vi "3kButtonsSys36x36.vi"() -> ()   [LabVIEW 2011]
doc: "3000 buttons from haobo.li@pansino.com.cn\nhttp://www.linkedin.com/pub/haobo-li/17/8a/220\nthanks to\nhttp://www.fatcow.com/free-icons"
panel:
  in  "Pansino 2":bool
  in  "Pansino":bool
  in  "zootool":bool
  in  "zoom_selection":bool
  in  "zoom_refresh":bool
  in  "zoom_out":bool
  in  "zoom_layer":bool
  in  "zoom_last":bool
  in  "zoom_in":bool
  in  "zoom_fit":bool
  in  "zoom_extend":bool
  in  "zoom_actual_equal":bool
  in  "zoom_actual":bool
  in  "zoom":bool
  in  "youtube":bool
  in  "yelp":bool
  in  "yellow_submarine":bool
  in  "yahoo_messenger":bool
  in  "yacht":bool
  in  "xing":bool
  in  "xhtml_valid":bool
  in  "xhtml_go":bool
  in  "xhtml_delete":bool
  in  "xhtml_add":bool
  in  "xhtml":bool
  in  "x_ray":bool
  in  "www_page":bool
  in  "wrench_orange":bool
  in  "wrench":bool
  in  "wrapping_tight":bool
  in  "wrapping_square":bool
  in  "wrapping_magazine":bool
  in  "wrapping_inline":bool
  in  "wrapping_in_front":bool
  in  "wrapping_edit":bool
  in  "wrapping_between":bool
  in  "wrapping_behind":bool
  in  "world_link":bool
  in  "world_go":bool
  in  "world_edit":bool
  in  "world_delete":bool
  in  "world_add":bool
  in  "world":bool
  in  "workspace":bool
  in  "wordpress_blog":bool
  in  "wordpress":bool
  in  "wizard_women":bool
  in  "wizard":bool
  in  "wishlist_add":bool
  in  "winrar_view":bool
  in  "winrar_extract":bool
  in  "winrar_add":bool
  in  "wine_pairings":bool
  in  "windy":bool
  in  "widgets":bool
  in  "widescreen":bool
  in  "whistle":bool
  in  "weight":bool
  in  "weighing_mashine":bool
  in  "webcam_error":bool
  in  "webcam_delete":bool
  in  "webcam_add":bool
  in  "webcam":bool
  in  "web_concierge":bool
  in  "weather_sun":bool
  in  "weather_snow":bool
  in  "weather_rain":bool
  in  "weather_lightning":bool
  in  "weather_cloudy":bool
  in  "weather_clouds":bool
  in  "wand":bool
  in  "wallet":bool
  in  "walk":bool
  in  "vslider":bool
  in  "vrule":bool
  in  "vlc":bool
  in  "visa_electron":bool
  in  "visa_2":bool
  in  "visa":bool
  in  "virus_protection":bool
  in  "virb":bool
  in  "vimeo":bool
  in  "viewstack":bool
  in  "videodisplay":bool
  in  "video_mode":bool
  in  "video":bool
  in  "viddler":bool
  in  "vhs":bool
  in  "vector_delete":bool
  in  "vector_add":bool
  in  "vector":bool
  in  "vdividedbox":bool
  in  "vcard_edit":bool
  in  "vcard_delete":bool
  in  "vcard_add":bool
  in  "vcard":bool
  in  "vbox":bool
  in  "user_zorro":bool
  in  "user_yoda":bool
  in  "user_wicket":bool
  in  "user_waiter_female_black":bool
  in  "user_waiter_female":bool
  in  "user_waiter":bool
  in  "user_viking_female":bool
  in  "user_viking":bool
  in  "user_vietnamese_female":bool
  in  "user_vietnamese":bool
  in  "user_trooper_captain":bool
  in  "user_trooper":bool
  in  "user_swimmer_female":bool
  in  "user_swimmer_black":bool
  in  "user_swimmer":bool
  in  "user_superman":bool
  in  "user_suit":bool
  in  "user_student_female_black":bool
  in  "user_student_female":bool
  in  "user_student_black":bool
  in  "user_student":bool
  in  "user_striper_black":bool
  in  "user_striper":bool
  in  "user_stewardess_black":bool
  in  "user_stewardess":bool
  in  "user_squidward":bool
  in  "user_sponge_bob":bool
  in  "user_spiderman":bool
  in  "user_soldier":bool
  in  "user_silhouette":bool
  in  "user_scream":bool
  in  "user_samurai":bool
  in  "user_sailor_black":bool
  in  "user_sailor":bool
  in  "user_robocop":bool
  in  "user_redskin":bool
  in  "user_red":bool
  in  "user_rambo":bool
  in  "user_racer":bool
  in  "user_r2d2":bool
  in  "user_queen_black":bool
  in  "user_queen":bool
  in  "user_pumpkin":bool
  in  "user_priest_black":bool
  in  "user_priest":bool
  in  "user_policeman_black":bool
  in  "user_policeman":bool
  in  "user_police_female_black":bool
  in  "user_police_female":bool
  in  "user_police_england":bool
  in  "user_plankton":bool
  in  "user_pirate":bool
  in  "user_pilot_civil":bool
  in  "user_pilot":bool
  in  "user_patrick":bool
  in  "user_orange":bool
  in  "user_oldwoman_black":bool
  in  "user_oldwoman":bool
  in  "user_oldman_black":bool
  in  "user_oldman":bool
  in  "user_officer_black":bool
  in  "user_officer":bool
  in  "user_nun_black":bool
  in  "user_nun":bool
  in  "user_nude_female_black":bool
  in  "user_nude_female":bool
  in  "user_nude_black":bool
  in  "user_nude":bool
  in  "user_ninja":bool
  in  "user_muslim_female":bool
  in  "user_muslim":bool
  in  "user_mexican":bool
  in  "user_medical_female_black":bool
  in  "user_medical_female":bool
  in  "user_medical_black":bool
  in  "user_medical":bool
  in  "user_maid":bool
  in  "user_lisa":bool
  in  "user_leprechaun":bool
  in  "user_knight":bool
  in  "user_king_black":bool
  in  "user_king":bool
  in  "user_judge_black":bool
  in  "user_judge":bool
  in  "user_jew":bool
  in  "user_jester":bool
  in  "user_jawa":bool
  in  "user_jason":bool
  in  "user_ironman":bool
  in  "user_indian_female":bool
  in  "user_indian":bool
  in  "user_imprisoned_female_black":bool
  in  "user_imprisoned_female":bool
  in  "user_imprisoned_black":bool
  in  "user_imprisoned":bool
  in  "user_hendrix":bool
  in  "user_halk":bool
  in  "user_green":bool
  in  "user_gray":bool
  in  "user_goth":bool
  in  "user_gomer":bool
  in  "user_go":bool
  in  "user_gladiator":bool
  in  "user_geisha":bool
  in  "user_freddy":bool
  in  "user_firefighter_black":bool
  in  "user_firefighter":bool
  in  "user_female":bool
  in  "user_eskimo_female":bool
  in  "user_eskimo":bool
  in  "user_emo":bool
  in  "user_egyptian_female":bool
  in  "user_egyptian":bool
  in  "user_edit":bool
  in  "user_dracula":bool
  in  "user_diver":bool
  in  "user_devil":bool
  in  "user_detective_gray":bool
  in  "user_detective":bool
  in  "user_delete":bool
  in  "user_death":bool
  in  "user_darth_vader":bool
  in  "user_crabs":bool
  in  "user_cowboy_female":bool
  in  "user_cowboy":bool
  in  "user_cook_female_black":bool
  in  "user_cook_female":bool
  in  "user_cook_black":bool
  in  "user_cook":bool
  in  "user_comment":bool
  in  "user_clown":bool
  in  "user_chief_female_black":bool
  in  "user_chief_female":bool
  in  "user_chief_black":bool
  in  "user_chief":bool
  in  "user_catwomen":bool
  in  "user_c3po":bool
  in  "user_buddhist":bool
  in  "user_boxer_black":bool
  in  "user_boxer":bool
  in  "user_blondy":bool
  in  "user_bishop":bool
  in  "user_bender":bool
  in  "user_beach_lifeguard_female":bool
  in  "user_beach_lifeguard":bool
  in  "user_batman":bool
  in  "user_bart":bool
  in  "user_banker":bool
  in  "user_ballplayer_black":bool
  in  "user_ballplayer":bool
  in  "user_astronaut":bool
  in  "user_angel_female_black":bool
  in  "user_angel_female":bool
  in  "user_angel_black":bool
  in  "user_angel":bool
  in  "user_alien":bool
  in  "user_add":bool
  in  "user":bool
  in  "usb_3":bool
  in  "update":bool
  in  "universal_binary":bool
  in  "unicorn":bool
  in  "understanding":bool
  in  "underle_dictionary":bool
  in  "umbrella":bool
  in  "ufo":bool
  in  "ubuntu":bool
  in  "twitter_2":bool
  in  "twitter_1":bool
  in  "tux":bool
  in  "turntable":bool
  in  "tumblr":bool
  in  "tubes":bool
  in  "tub":bool
  in  "trolley":bool
  in  "trojan_horse":bool
  in  "tree":bool
  in  "travel":bool
  in  "transmit_go":bool
  in  "transmit_error":bool
  in  "transmit_edit":bool
  in  "transmit_delete":bool
  in  "transmit_blue":bool
  in  "transmit_add":bool
  in  "transmit":bool
  in  "transform_shear":bool
  in  "transform_selection":bool
  in  "transform_scale":bool
  in  "transform_rotate_270":bool
  in  "transform_rotate_180":bool
  in  "transform_rotate_90":bool
  in  "transform_rotate":bool
  in  "transform_perspective":bool
  in  "transform_path":bool
  in  "transform_move":bool
  in  "transform_layer":bool
  in  "transform_flip":bool
  in  "transform_crop_resize":bool
  in  "transform_crop":bool
  in  "traffic_usage":bool
  in  "traffic_lights_yellow":bool
  in  "traffic_lights_red":bool
  in  "traffic_lights_green":bool
  in  "traffic_lights":bool
  in  "trade":bool
  in  "tractor":bool
  in  "toxic":bool
  in  "tower":bool
  in  "toucan":bool
  in  "total_plan_cost":bool
  in  "toster":bool
  in  "tornado":bool
  in  "torchere":bool
  in  "tooth":bool
  in  "toolbox":bool
  in  "to_do_list_cheked_all":bool
  in  "to_do_list_cheked_1":bool
  in  "to_do_list":bool
  in  "title_window":bool
  in  "tire":bool
  in  "tipper":bool
  in  "timeline_marker":bool
  in  "timeline":bool
  in  "time_go":bool
  in  "time_delete":bool
  in  "time_add":bool
  in  "time":bool
  in  "tilelist":bool
  in  "tick":bool
  in  "thumb_up":bool
  in  "thumb_down":bool
  in  "three_tags":bool
  in  "things_digital":bool
  in  "things_beauty":bool
  in  "theater":bool
  in  "textfield_rename":bool
  in  "textfield_key":bool
  in  "textfield_delete":bool
  in  "textfield_add":bool
  in  "textfield":bool
  in  "text_width":bool
  in  "text_uppercase":bool
  in  "text_underline":bool
  in  "text_superscript":bool
  in  "text_subscript":bool
  in  "text_strikethroungh":bool
  in  "text_smallcaps":bool
  in  "text_signature":bool
  in  "text_resize":bool
  in  "text_replace":bool
  in  "text_prose":bool
  in  "text_pagination_100":bool
  in  "text_pagination":bool
  in  "text_padding_top":bool
  in  "text_padding_right":bool
  in  "text_padding_left":bool
  in  "text_padding_bottom":bool
  in  "text_lowercase":bool
  in  "text_list_numbers":bool
  in  "text_list_bullets":bool
  in  "text_linespacing":bool
  in  "text_letterspacing":bool
  in  "text_letter_omega":bool
  in  "text_large_cap":bool
  in  "text_language":bool
  in  "text_kerning":bool
  in  "text_italic":bool
  in  "text_indent_remove":bool
  in  "text_indent":bool
  in  "text_horizontalrule":bool
  in  "text_heading_6":bool
  in  "text_heading_5":bool
  in  "text_heading_4":bool
  in  "text_heading_3":bool
  in  "text_heading_2":bool
  in  "text_heading_1":bool
  in  "text_dropcaps":bool
  in  "text_drama":bool
  in  "text_document_wrap":bool
  in  "text_document":bool
  in  "text_columns":bool
  in  "text_bold":bool
  in  "text_area":bool
  in  "text_allcaps":bool
  in  "text_align_right":bool
  in  "text_align_left":bool
  in  "text_align_justity":bool
  in  "text_align_center":bool
  in  "text":bool
  in  "terminal_seats_red":bool
  in  "terminal_seats_blue":bool
  in  "terminal":bool
  in  "temperature_5":bool
  in  "temperature_4":bool
  in  "temperature_3":bool
  in  "temperature_2":bool
  in  "temperature_1":bool
  in  "television_delete":bool
  in  "television_add":bool
  in  "television":bool
  in  "telephone_link":bool
  in  "telephone_key":bool
  in  "telephone_go":bool
  in  "telephone_error":bool
  in  "telephone_edit":bool
  in  "telephone_delete":bool
  in  "telephone_add":bool
  in  "telephone":bool
  in  "teddy_bear":bool
  in  "technorati":bool
  in  "teapot":bool
  in  "tea_cup":bool
  in  "tags_cloud":bool
  in  "tag_yellow":bool
  in  "tag_red":bool
  in  "tag_purple":bool
  in  "tag_pink":bool
  in  "tag_orange":bool
  in  "tag_green":bool
  in  "tag_blue_edit":bool
  in  "tag_blue_delete":bool
  in  "tag_blue_add":bool
  in  "tag_blue":bool
  in  "tag":bool
  in  "tabnavigator":bool
  in  "tablets":bool
  in  "table_torn":bool
  in  "table_tab_search":bool
  in  "table_tab_resize":bool
  in  "table_tab":bool
  in  "table_sum":bool
  in  "table_split":bool
  in  "table_sort":bool
  in  "table_sheet":bool
  in  "table_select_row":bool
  in  "table_select_column":bool
  in  "table_select_big":bool
  in  "table_select_all":bool
  in  "table_select":bool
  in  "table_save":bool
  in  "table_row_insert":bool
  in  "table_row_delete":bool
  in  "table_replace":bool
  in  "table_relationship":bool
  in  "table_refresh":bool
  in  "table_paint_can":bool
  in  "table_multiple":bool
  in  "table_money":bool
  in  "table_link":bool
  in  "table_lightning":bool
  in  "table_key":bool
  in  "table_insert":bool
  in  "table_import":bool
  in  "table_heatmap":bool
  in  "table_go":bool
  in  "table_gear":bool
  in  "table_export":bool
  in  "table_excel":bool
  in  "table_error":bool
  in  "table_edit":bool
  in  "table_delete":bool
  in  "table_chart":bool
  in  "table_add":bool
  in  "table":bool
  in  "tabbar":bool
  in  "tab_go":bool
  in  "tab_edit":bool
  in  "tab_delete":bool
  in  "tab_add":bool
  in  "tab":bool
  in  "system_time":bool
  in  "system_monitor":bool
  in  "sword":bool
  in  "switch_220v":bool
  in  "switch_120v":bool
  in  "switch":bool
  in  "swf_loader":bool
  in  "support":bool
  in  "sun_rain":bool
  in  "sun_cloudy":bool
  in  "sum":bool
  in  "subwoofer":bool
  in  "style_go":bool
  in  "style_edit":bool
  in  "style_delete":bool
  in  "style_add":bool
  in  "style":bool
  in  "stumble_upon":bool
  in  "street_stall":bool
  in  "storage":bool
  in  "stopwatch_start":bool
  in  "stopwatch_pause":bool
  in  "stopwatch_finish":bool
  in  "stop":bool
  in  "stethoscope_vintage":bool
  in  "stethoscope":bool
  in  "steering_wheel_3":bool
  in  "steering_wheel_2":bool
  in  "steering_wheel":bool
  in  "steak_meat":bool
  in  "steak_fish":bool
  in  "status_online":bool
  in  "status_offline":bool
  in  "status_busy":bool
  in  "status_away":bool
  in  "statistics":bool
  in  "star":bool
  in  "stamp_pattern":bool
  in  "ssl_certificates":bool
  in  "sql_join_right_exclude":bool
  in  "sql_join_right":bool
  in  "sql_join_outer_exclude":bool
  in  "sql_join_outer":bool
  in  "sql_join_left_exclude":bool
  in  "sql_join_left":bool
  in  "sql_join_inner":bool
  in  "sql_join":bool
  in  "spring":bool
  in  "sport_tennis":bool
  in  "sport_soccer":bool
  in  "sport_shuttlecock":bool
  in  "sport_raquet":bool
  in  "sport_golf":bool
  in  "sport_football":bool
  in  "sport_basketball":bool
  in  "sport_8ball":bool
  in  "sport":bool
  in  "spill":bool
  in  "spider_web":bool
  in  "spellcheck_error":bool
  in  "spellcheck":bool
  in  "speedometer":bool
  in  "speakers":bool
  in  "spam_filter":bool
  in  "spam":bool
  in  "spacer":bool
  in  "source_code":bool
  in  "soup":bool
  in  "sound_none":bool
  in  "sound_mute":bool
  in  "sound_low":bool
  in  "sound_delete":bool
  in  "sound_add":bool
  in  "sound":bool
  in  "sort_descending":bool
  in  "sort_columns":bool
  in  "sort_ascending":bool
  in  "solar":bool
  in  "soil_layers":bool
  in  "soap":bool
  in  "snowman":bool
  in  "snow_rain":bool
  in  "sneakers":bool
  in  "snapshot":bool
  in  "snake_and_cup":bool
  in  "snail":bool
  in  "small_tiles":bool
  in  "small_car":bool
  in  "small_business":bool
  in  "slideshow":bool
  in  "slackware":bool
  in  "skype":bool
  in  "skins":bool
  in  "skate":bool
  in  "size_vertical":bool
  in  "size_horizontal":bool
  in  "sitemap_color":bool
  in  "sitemap":bool
  in  "site_enhancer":bool
  in  "site_backup_and_restore":bool
  in  "siren":bool
  in  "sign":bool
  in  "shuriken":bool
  in  "showel":bool
  in  "shorts":bool
  in  "shopping":bool
  in  "shop_open":bool
  in  "shop_closed":bool
  in  "shirt_polo":bool
  in  "shield_go":bool
  in  "shield_delete":bool
  in  "shield_add":bool
  in  "shield":bool
  in  "sheduled_task":bool
  in  "sharpen":bool
  in  "share":bool
  in  "shape_ungroup":bool
  in  "shape_square_link":bool
  in  "shape_square_key":bool
  in  "shape_square_go":bool
  in  "shape_square_error":bool
  in  "shape_square_edit":bool
  in  "shape_square_delete":bool
  in  "shape_square_add":bool
  in  "shape_square":bool
  in  "shape_rotate_clockwise":bool
  in  "shape_rotate_anticlockwise":bool
  in  "shape_move_front":bool
  in  "shape_move_forwards":bool
  in  "shape_move_backwards":bool
  in  "shape_move_back":bool
  in  "shape_handles":bool
  in  "shape_group":bool
  in  "shape_flip_vertical":bool
  in  "shape_flip_horizontal":bool
  in  "shape_align_top":bool
  in  "shape_align_right":bool
  in  "shape_align_middle":bool
  in  "shape_align_left":bool
  in  "shape_align_center":bool
  in  "shape_align_bottom":bool
  in  "shading":bool
  in  "setting_tools":bool
  in  "set_security_question":bool
  in  "session_idle_time":bool
  in  "server_uncompress":bool
  in  "server_stanchion":bool
  in  "server_link":bool
  in  "server_lightning":bool
  in  "server_key":bool
  in  "server_information":bool
  in  "server_go":bool
  in  "server_error":bool
  in  "server_edit":bool
  in  "server_delete":bool
  in  "server_database":bool
  in  "server_connect":bool
  in  "server_compress":bool
  in  "server_components":bool
  in  "server_chart":bool
  in  "server_add":bool
  in  "server":bool
  in  "sertificate":bool
  in  "select_restangular":bool
  in  "select_lasso":bool
  in  "select_invert":bool
  in  "select_ellipse":bool
  in  "select_continuous_area":bool
  in  "select_by_intersection":bool
  in  "select_by_difference":bool
  in  "select_by_color":bool
  in  "select_by_adding_to_selection":bool
  in  "select":bool
  in  "search_plus":bool
  in  "search_minus":bool
  in  "scull":bool
  in  "scroller_bar":bool
  in  "scripts":bool
  in  "script_yellow":bool
  in  "script_torn":bool
  in  "script_save":bool
  in  "script_red":bool
  in  "script_palette":bool
  in  "script_link":bool
  in  "script_lightning":bool
  in  "script_key":bool
  in  "script_green":bool
  in  "script_go":bool
  in  "script_gear":bool
  in  "script_error":bool
  in  "script_edit":bool
  in  "script_delete":bool
  in  "script_code_red":bool
  in  "script_code":bool
  in  "script_black":bool
  in  "script_add":bool
  in  "script":bool
  in  "screwdriver":bool
  in  "screen_error":bool
  in  "scanner":bool
  in  "scalpel":bool
  in  "scale_image":bool
  in  "save_money":bool
  in  "save_as":bool
  in  "satellite_dish":bool
  in  "satellite":bool
  in  "santa":bool
  in  "salver":bool
  in  "sallary_deferrais":bool
  in  "safe":bool
  in  "safari_browser":bool
  in  "ruby_put":bool
  in  "ruby_link":bool
  in  "ruby_key":bool
  in  "ruby_go":bool
  in  "ruby_get":bool
  in  "ruby_gear":bool
  in  "ruby_delete":bool
  in  "ruby_add":bool
  in  "ruby":bool
  in  "rubber_duck":bool
  in  "rss_valid":bool
  in  "rss_go":bool
  in  "rss_delete":bool
  in  "rss_add":bool
  in  "rss":bool
  in  "routing_turning_right":bool
  in  "routing_turning_left":bool
  in  "routing_turnaround_right":bool
  in  "routing_turnaround_left":bool
  in  "routing_turn_u":bool
  in  "routing_turn_right_2":bool
  in  "routing_turn_right":bool
  in  "routing_turn_left_crossroads":bool
  in  "routing_turn_left_2":bool
  in  "routing_turn_left":bool
  in  "routing_turn_arround_right":bool
  in  "routing_turn_arround_left":bool
  in  "routing_intersection_right":bool
  in  "routing_go_straight_right":bool
  in  "routing_go_straight_left":bool
  in  "routing_go_right":bool
  in  "routing_go_left":bool
  in  "routing_forward":bool
  in  "routing_around":bool
  in  "router":bool
  in  "rotate_90":bool
  in  "rosette":bool
  in  "role":bool
  in  "rocking_chair":bool
  in  "robo_to":bool
  in  "roadworks":bool
  in  "road_sign":bool
  in  "rip":bool
  in  "ring":bool
  in  "richtext_editor":bool
  in  "ribbon":bool
  in  "resultset_previous":bool
  in  "resultset_next":bool
  in  "resultset_last":bool
  in  "resultset_first":bool
  in  "restaurant_menu":bool
  in  "resources":bool
  in  "resource_usage":bool
  in  "resize_picture":bool
  in  "reseller_programm":bool
  in  "reseller_account_template":bool
  in  "reseller_account":bool
  in  "report_word":bool
  in  "report_user":bool
  in  "report_torn":bool
  in  "report_picture":bool
  in  "report_magnify":bool
  in  "report_link":bool
  in  "report_key":bool
  in  "report_go":bool
  in  "report_edit":bool
  in  "report_disk":bool
  in  "report_delete":bool
  in  "report_add":bool
  in  "report":bool
  in  "remote":bool
  in  "reddit":bool
  in  "red_line":bool
  in  "recycle_bag":bool
  in  "recycle":bool
  in  "real_estate":bool
  in  "readernaut":bool
  in  "rainbow_cloud":bool
  in  "rainbow":bool
  in  "rain":bool
  in  "radiolocator":bool
  in  "radiobutton_group":bool
  in  "radiobutton":bool
  in  "radioactivity":bool
  in  "radio_2":bool
  in  "radio_1":bool
  in  "rabbit":bool
  in  "question":bool
  in  "qip_online":bool
  in  "qip_offline":bool
  in  "qip_occupied":bool
  in  "qip_not_available":bool
  in  "qip_invisible_for_all":bool
  in  "qip_invisible":bool
  in  "qip_free_for_chat":bool
  in  "qip_eating":bool
  in  "qip_dnd":bool
  in  "qip_bad_mood":bool
  in  "qip_away":bool
  in  "qip_at_work":bool
  in  "qip_at_home":bool
  in  "qip_angry":bool
  in  "qik":bool
  in  "purse":bool
  in  "progressbar":bool
  in  "profiles":bool
  in  "production_copyleft":bool
  in  "processor":bool
  in  "private":bool
  in  "printer_error":bool
  in  "printer_empty":bool
  in  "printer_delete":bool
  in  "printer_add":bool
  in  "printer":bool
  in  "print_size":bool
  in  "price_watch":bool
  in  "price_comparison":bool
  in  "price_alert":bool
  in  "premium_support":bool
  in  "preferences":bool
  in  "power_surge":bool
  in  "posterous":bool
  in  "postage_stamp":bool
  in  "port":bool
  in  "popcorn":bool
  in  "pop_mail":bool
  in  "poo":bool
  in  "poker":bool
  in  "plurk":bool
  in  "plugin_link":bool
  in  "plugin_go":bool
  in  "plugin_error":bool
  in  "plugin_edit":bool
  in  "plugin_disabled":bool
  in  "plugin_delete":bool
  in  "plugin_add":bool
  in  "plugin":bool
  in  "plotchart":bool
  in  "playstation":bool
  in  "Plant":bool
  in  "plane":bool
  in  "places":bool
  in  "pizza":bool
  in  "pirate_flag":bool
  in  "pint":bool
  in  "pill_go":bool
  in  "pill_delete":bool
  in  "pill_add":bool
  in  "pill":bool
  in  "pilcrow":bool
  in  "piechart":bool
  in  "piece_of_cake":bool
  in  "pictures":bool
  in  "picture_save":bool
  in  "picture_link":bool
  in  "picture_key":bool
  in  "picture_go":bool
  in  "picture_frame":bool
  in  "picture_error":bool
  in  "picture_empty":bool
  in  "picture_edit":bool
  in  "picture_delete":bool
  in  "picture_add":bool
  in  "picture":bool
  in  "picasa":bool
  in  "piano":bool
  in  "pi_math":bool
  in  "photos":bool
  in  "photo_link":bool
  in  "photo_delete":bool
  in  "photo_add":bool
  in  "photo":bool
  in  "phone_vintage":bool
  in  "phone_sound":bool
  in  "phone_delete":bool
  in  "phone_Android":bool
  in  "phone_add":bool
  in  "phone":bool
  in  "personals":bool
  in  "personal_finance":bool
  in  "perfomance":bool
  in  "pepper":bool
  in  "pencil_go":bool
  in  "pencil_delete":bool
  in  "pencil_add":bool
  in  "pencil":bool
  in  "pearl":bool
  in  "peak_cap":bool
  in  "peacock":bool
  in  "pci":bool
  in  "pc_linux_os":bool
  in  "paypal-2":bool
  in  "paypal":bool
  in  "paste_word":bool
  in  "paste_plain":bool
  in  "participation_rate":bool
  in  "parrot":bool
  in  "paper_airplane":bool
  in  "panel":bool
  in  "pandora":bool
  in  "palette":bool
  in  "paintcan":bool
  in  "painbrush":bool
  in  "page_world":bool
  in  "page_word":bool
  in  "page_white_zip":bool
  in  "page_white_wrench":bool
  in  "page_white_world":bool
  in  "page_white_word":bool
  in  "page_white_width":bool
  in  "page_white_visualstudio":bool
  in  "page_white_vector":bool
  in  "page_white_tux":bool
  in  "page_white_text_width":bool
  in  "page_white_text":bool
  in  "page_white_star":bool
  in  "page_white_stack":bool
  in  "page_white_ruby":bool
  in  "page_white_put":bool
  in  "page_white_powerpoint":bool
  in  "page_white_picture":bool
  in  "page_white_php":bool
  in  "page_white_paste":bool
  in  "page_white_paintbrush":bool
  in  "page_white_paint":bool
  in  "page_white_office":bool
  in  "page_white_medal":bool
  in  "page_white_magnify":bool
  in  "page_white_link":bool
  in  "page_white_lightning":bool
  in  "page_white_key":bool
  in  "page_white_horizontal":bool
  in  "page_white_h":bool
  in  "page_white_go":bool
  in  "page_white_get":bool
  in  "page_white_gear":bool
  in  "page_white_flash":bool
  in  "page_white_find":bool
  in  "page_white_excel":bool
  in  "page_white_error":bool
  in  "page_white_edit":bool
  in  "page_white_dvd":bool
  in  "page_white_delete":bool
  in  "page_white_database":bool
  in  "page_white_cup":bool
  in  "page_white_csharp":bool
  in  "page_white_cplusplus":bool
  in  "page_white_copy":bool
  in  "page_white_compress":bool
  in  "page_white_code_red":bool
  in  "page_white_code":bool
  in  "page_white_cd":bool
  in  "page_white_camera":bool
  in  "page_white_c":bool
  in  "page_white_add":bool
  in  "page_white_actionscript":bool
  in  "page_white_acrobat":bool
  in  "page_white":bool
  in  "page_save":bool
  in  "page_refresh":bool
  in  "page_red":bool
  in  "page_paste":bool
  in  "page_paintbrush":bool
  in  "page_magnifier":bool
  in  "page_link":bool
  in  "page_lightning":bool
  in  "page_key":bool
  in  "page_green":bool
  in  "page_go":bool
  in  "page_gear":bool
  in  "page_find":bool
  in  "page_excel":bool
  in  "page_error":bool
  in  "page_edit":bool
  in  "page_delete":bool
  in  "page_copy":bool
  in  "page_code":bool
  in  "page_attach":bool
  in  "page_add":bool
  in  "page":bool
  in  "package_link":bool
  in  "package_green":bool
  in  "package_go":bool
  in  "package_delete":bool
  in  "package_add":bool
  in  "package":bool
  in  "other_phone":bool
  in  "orthodox_church":bool
  in  "ornament_gold":bool
  in  "orkut":bool
  in  "origami":bool
  in  "orbit":bool
  in  "opera":bool
  in  "openid":bool
  in  "open_suse":bool
  in  "open_folder":bool
  in  "omelet":bool
  in  "oil":bool
  in  "numeric_stepper":bool
  in  "note_torn":bool
  in  "note_go":bool
  in  "note_error":bool
  in  "note_edit":bool
  in  "note_delete":bool
  in  "note_add":bool
  in  "note":bool
  in  "non_derivative":bool
  in  "nokia_s60":bool
  in  "node-tree":bool
  in  "no_smoking":bool
  in  "no_requirements":bool
  in  "no_image":bool
  in  "no_drm_trm":bool
  in  "no_commercial":bool
  in  "newsvine":bool
  in  "newspaper_link":bool
  in  "newspaper_go":bool
  in  "newspaper_delete":bool
  in  "newspaper_add":bool
  in  "newspaper":bool
  in  "new":bool
  in  "network-share":bool
  in  "networking_red":bool
  in  "networking_green":bool
  in  "networking":bool
  in  "network_wireless":bool
  in  "network_ip":bool
  in  "network_hub":bool
  in  "network_folder":bool
  in  "network_firewall":bool
  in  "network_ethernet":bool
  in  "network_clouds":bool
  in  "network_cloud":bool
  in  "network_adapter":bool
  in  "netvibes":bool
  in  "nameboard_open":bool
  in  "myspace":bool
  in  "my_name_is_e":bool
  in  "mustache":bool
  in  "music":bool
  in  "multitool":bool
  in  "multiplied_by_100":bool
  in  "multiplied_by_10":bool
  in  "multiplied_by_5":bool
  in  "multiplied_by_3":bool
  in  "multiplied_by_2":bool
  in  "msn_messenger":bool
  in  "ms_frontpage":bool
  in  "ms_exchange":bool
  in  "movies":bool
  in  "move_to_folder":bool
  in  "mouse_select_scroll":bool
  in  "mouse_select_right":bool
  in  "mouse_select_left":bool
  in  "mouse_error":bool
  in  "mouse_delete":bool
  in  "mouse_add":bool
  in  "mouse_2":bool
  in  "mouse":bool
  in  "motherboard":bool
  in  "mosque":bool
  in  "moon":bool
  in  "monitor_window_3d":bool
  in  "monitor_window":bool
  in  "monitor_wallpaper":bool
  in  "monitor_sidebar":bool
  in  "monitor_screensaver":bool
  in  "monitor_link":bool
  in  "monitor_lightning":bool
  in  "monitor_go":bool
  in  "monitor_error":bool
  in  "monitor_edit":bool
  in  "monitor_delete":bool
  in  "monitor_add":bool
  in  "monitor":bool
  in  "moneybox":bool
  in  "money_yen":bool
  in  "money_pound":bool
  in  "money_in_envelope":bool
  in  "money_euro":bool
  in  "money_dollar":bool
  in  "money_delete":bool
  in  "money_bookers":bool
  in  "money_bag":bool
  in  "money_add":bool
  in  "money":bool
  in  "molecule":bool
  in  "mobile_me":bool
  in  "mixx":bool
  in  "mixture":bool
  in  "mixer":bool
  in  "milestone":bool
  in  "microwave":bool
  in  "microscope":bool
  in  "microphone":bool
  in  "microformats":bool
  in  "micro_sd_blue":bool
  in  "micro_sd":bool
  in  "metronome":bool
  in  "metro":bool
  in  "messenger":bool
  in  "menubar":bool
  in  "menu_item":bool
  in  "menu":bool
  in  "medical_record":bool
  in  "medal_silver_delete":bool
  in  "medal_silver_add":bool
  in  "medal_silver_3":bool
  in  "medal_silver_2":bool
  in  "medal_silver_1":bool
  in  "medal_gold_delete":bool
  in  "medal_gold_add":bool
  in  "medal_gold_3":bool
  in  "medal_gold_2":bool
  in  "medal_gold_1":bool
  in  "medal_bronze_delete":bool
  in  "medal_bronze_add":bool
  in  "medal_bronze_3":bool
  in  "medal_bronze_2":bool
  in  "medal_bronze_1":bool
  in  "medal_award_silver":bool
  in  "medal_award_gold":bool
  in  "medal_award_bronze":bool
  in  "measure_crop":bool
  in  "measure":bool
  in  "master_card":bool
  in  "mask":bool
  in  "marketwatch":bool
  in  "mario":bool
  in  "map_torn":bool
  in  "map_magnify":bool
  in  "map_go":bool
  in  "map_edit":bool
  in  "map_delete":bool
  in  "map_add":bool
  in  "map":bool
  in  "mandriva":bool
  in  "male":bool
  in  "mail-trash":bool
  in  "mail_yellow":bool
  in  "mail_torn":bool
  in  "mail_server_setting":bool
  in  "mail_red":bool
  in  "mail_green":bool
  in  "mail_box":bool
  in  "mail_black":bool
  in  "magnifier_zoom_out":bool
  in  "magnifier_zoom_in":bool
  in  "magnifier":bool
  in  "magnet":bool
  in  "magic_wand_2":bool
  in  "luggage_brown_tag":bool
  in  "luggage_brown":bool
  in  "luggage":bool
  in  "lorry_link":bool
  in  "lorry_go":bool
  in  "lorry_flatbed":bool
  in  "lorry_error":bool
  in  "lorry_delete":bool
  in  "lorry_add":bool
  in  "lorry":bool
  in  "lollypop":bool
  in  "lollipop":bool
  in  "lock_open":bool
  in  "lock_go":bool
  in  "lock_edit":bool
  in  "lock_delete":bool
  in  "lock_break":bool
  in  "lock_add":bool
  in  "lock":bool
  in  "location_pin":bool
  in  "locate":bool
  in  "livejournal":bool
  in  "list":bool
  in  "linux_mint":bool
  in  "linkedin":bool
  in  "linkbar":bool
  in  "link_unchain":bool
  in  "link_juice":bool
  in  "link_go":bool
  in  "link_edit":bool
  in  "link_delete":bool
  in  "link_button":bool
  in  "link_break":bool
  in  "link_add":bool
  in  "link":bool
  in  "linechart":bool
  in  "line_split":bool
  in  "lightning_go":bool
  in  "lightning_delete":bool
  in  "lightning_add":bool
  in  "lightning":bool
  in  "lighthouse_shine":bool
  in  "lighthouse":bool
  in  "lightbulb_off":bool
  in  "lightbulb_delete":bool
  in  "lightbulb_add":bool
  in  "lightbulb":bool
  in  "light_circle_green":bool
  in  "life_vest":bool
  in  "license_management":bool
  in  "license_key":bool
  in  "legend":bool
  in  "led":bool
  in  "layouts_split_vertical":bool
  in  "layouts_split":bool
  in  "layouts_select_sidebar":bool
  in  "layouts_select_footer":bool
  in  "layouts_select_content":bool
  in  "layouts_select":bool
  in  "layouts_join_vertical":bool
  in  "layouts_join":bool
  in  "layouts_hf_3":bool
  in  "layouts_hf_2_equal":bool
  in  "layouts_header_footer_3":bool
  in  "layouts_header_footer_2":bool
  in  "layouts_header_footer":bool
  in  "layouts_header_3_mix":bool
  in  "layouts_header_3":bool
  in  "layouts_header_2_equal":bool
  in  "layouts_header_2":bool
  in  "layouts_header":bool
  in  "layouts_design":bool
  in  "layouts_6":bool
  in  "layouts_4":bool
  in  "layouts_3_mix":bool
  in  "layouts_3":bool
  in  "layouts_2":bool
  in  "layouts":bool
  in  "layout_sidebar":bool
  in  "layout_link":bool
  in  "layout_header":bool
  in  "layout_error":bool
  in  "layout_edit":bool
  in  "layout_delete":bool
  in  "layout_content":bool
  in  "layout_add":bool
  in  "layout":bool
  in  "layers_map":bool
  in  "layers":bool
  in  "layer_wms":bool
  in  "layer_vector":bool
  in  "layer_transparent":bool
  in  "layer_to_image_size":bool
  in  "layer_stack_arrange_back":bool
  in  "layer_stack_arrange":bool
  in  "layer_shred":bool
  in  "layer_shape_text":bool
  in  "layer_shape_round":bool
  in  "layer_shape_polyline":bool
  in  "layer_shape_ellipse":bool
  in  "layer_shape":bool
  in  "layer_shaded_relief":bool
  in  "layer_shade":bool
  in  "layer_select":bool
  in  "layer_save":bool
  in  "layer_rgb":bool
  in  "layer_resize_replicate_v":bool
  in  "layer_resize_replicate_h":bool
  in  "layer_resize_actual":bool
  in  "layer_resize":bool
  in  "layer_remove":bool
  in  "layer_redraw":bool
  in  "layer_raster_3d":bool
  in  "layer_raster":bool
  in  "layer_open":bool
  in  "layer_mask":bool
  in  "layer_label":bool
  in  "layer_import":bool
  in  "layer_histogram":bool
  in  "layer_his":bool
  in  "layer_group":bool
  in  "layer_grid":bool
  in  "layer_gps":bool
  in  "layer_export":bool
  in  "layer_edit":bool
  in  "layer_delete":bool
  in  "layer_database":bool
  in  "layer_create":bool
  in  "layer_command":bool
  in  "layer_chart":bool
  in  "layer_cell_cats":bool
  in  "layer_aspect_arrow":bool
  in  "layer_arrange_back":bool
  in  "layer_arrange":bool
  in  "layer_add":bool
  in  "layer":bool
  in  "last_fm":bool
  in  "large_tiles":bool
  in  "laptop":bool
  in  "language":bool
  in  "landmarks":bool
  in  "ladybird":bool
  in  "knot":bool
  in  "kids":bool
  in  "keyboard_magnify":bool
  in  "keyboard_delete":bool
  in  "keyboard_add":bool
  in  "keyboard":bool
  in  "key_z":bool
  in  "key_y":bool
  in  "key_x":bool
  in  "key_w":bool
  in  "key_v":bool
  in  "key_u":bool
  in  "key_t":bool
  in  "key_solid":bool
  in  "key_s":bool
  in  "key_r":bool
  in  "key_q":bool
  in  "key_p":bool
  in  "key_o":bool
  in  "key_n":bool
  in  "key_m":bool
  in  "key_l":bool
  in  "key_k":bool
  in  "key_j":bool
  in  "key_i":bool
  in  "key_h":bool
  in  "key_go":bool
  in  "key_g":bool
  in  "key_f":bool
  in  "key_escape":bool
  in  "key_e":bool
  in  "key_delete":bool
  in  "key_d":bool
  in  "key_c":bool
  in  "key_b":bool
  in  "key_add":bool
  in  "key_a":bool
  in  "key":bool
  in  "json":bool
  in  "joystick_error":bool
  in  "joystick_delete":bool
  in  "joystick_add":bool
  in  "joystick":bool
  in  "jeans":bool
  in  "jason_mask":bool
  in  "jar_open":bool
  in  "jar_empty":bool
  in  "jacket":bool
  in  "italy":bool
  in  "ipod_sound":bool
  in  "ipod_cast_delete":bool
  in  "ipod_cast_add":bool
  in  "ipod_cast":bool
  in  "ipod":bool
  in  "iphone":bool
  in  "ipad":bool
  in  "ip_class":bool
  in  "ip_block":bool
  in  "ip":bool
  in  "investment_menu_quality":bool
  in  "internet_explorer":bool
  in  "interface_preferences":bool
  in  "installer_box":bool
  in  "insert_object":bool
  in  "insert_element":bool
  in  "injection":bool
  in  "information":bool
  in  "info_rhombus":bool
  in  "index-cards":bool
  in  "inbox_upload":bool
  in  "inbox_table":bool
  in  "inbox_slide":bool
  in  "inbox_images":bool
  in  "inbox_film":bool
  in  "inbox_empty":bool
  in  "inbox_download":bool
  in  "inbox_document_text":bool
  in  "inbox_document_music":bool
  in  "inbox_document":bool
  in  "images_flickr":bool
  in  "images":bool
  in  "image_link":bool
  in  "image_edit":bool
  in  "image_delete":bool
  in  "image_add":bool
  in  "image":bool
  in  "im_messenger":bool
  in  "ilike":bool
  in  "icecream":bool
  in  "ice_cube":bool
  in  "hummingbird":bool
  in  "http_status_unavailable":bool
  in  "http_status_temporary":bool
  in  "http_status_server_error":bool
  in  "http_status_permanent":bool
  in  "http_status_ok_success":bool
  in  "http_status_not_found":bool
  in  "html_valid":bool
  in  "html_go":bool
  in  "html_delete":bool
  in  "html_add":bool
  in  "html_5":bool
  in  "html":bool
  in  "hslider":bool
  in  "hrule":bool
  in  "house_two":bool
  in  "house_one":bool
  in  "house_link":bool
  in  "house_go":bool
  in  "house":bool
  in  "hourglass_link":bool
  in  "hourglass_go":bool
  in  "hourglass_delete":bool
  in  "hourglass_add":bool
  in  "hourglass":bool
  in  "hotjobs":bool
  in  "hot":bool
  in  "hostname":bool
  in  "hospital":bool
  in  "horoscopes":bool
  in  "horn":bool
  in  "horizontal_list":bool
  in  "home_page":bool
  in  "holly":bool
  in  "hlocchart":bool
  in  "hippocampus":bool
  in  "highlighter_text":bool
  in  "highlighter":bool
  in  "help":bool
  in  "helmet_mine":bool
  in  "helmet":bool
  in  "helicopter":bool
  in  "heart_half":bool
  in  "heart_empty":bool
  in  "heart_delete":bool
  in  "heart_break":bool
  in  "heart_add":bool
  in  "heart":bool
  in  "health":bool
  in  "headphone_mic":bool
  in  "headphone":bool
  in  "hdividedbox":bool
  in  "hd_ready":bool
  in  "hd_1080":bool
  in  "hd_720":bool
  in  "hbox":bool
  in  "hat":bool
  in  "hardware_building_oem":bool
  in  "handbag":bool
  in  "hand_property":bool
  in  "hand_point_270":bool
  in  "hand_point_180":bool
  in  "hand_point_090":bool
  in  "hand_point":bool
  in  "hand_ily":bool
  in  "hand_fuck":bool
  in  "hand":bool
  in  "hammer":bool
  in  "hamburger":bool
  in  "half_moon":bool
  in  "gun":bool
  in  "group_link":bool
  in  "group_key":bool
  in  "group_go":bool
  in  "group_gear":bool
  in  "group_error":bool
  in  "group_edit":bool
  in  "group_delete":bool
  in  "group_add":bool
  in  "group":bool
  in  "grooveshark":bool
  in  "grid":bool
  in  "grenade":bool
  in  "green_yellow":bool
  in  "green_wormhole":bool
  in  "green":bool
  in  "grass":bool
  in  "gps_handheld":bool
  in  "gps_automotive":bool
  in  "gowalla":bool
  in  "google_webmaster_tools":bool
  in  "google_web_elements":bool
  in  "google_wave":bool
  in  "google_voice":bool
  in  "google_talk":bool
  in  "google_plus":bool
  in  "google_new":bool
  in  "google_map_satellite":bool
  in  "google_map":bool
  in  "google_custom_search":bool
  in  "google_adsense":bool
  in  "google":bool
  in  "globe_place":bool
  in  "globe_network":bool
  in  "globe_model":bool
  in  "global_telecom":bool
  in  "glass_narrow":bool
  in  "gift_add":bool
  in  "geotag":bool
  in  "georectify":bool
  in  "gentoo_linux":bool
  in  "gear_in":bool
  in  "gcp_rms":bool
  in  "gcp":bool
  in  "gas":bool
  in  "gamespot":bool
  in  "game_monitor":bool
  in  "ftp":bool
  in  "fruit_lime":bool
  in  "fruit_grape":bool
  in  "friendfeed":bool
  in  "freebsd":bool
  in  "forrst":bool
  in  "formheading":bool
  in  "form":bool
  in  "forklift":bool
  in  "font_superscript":bool
  in  "font_subscript":bool
  in  "font_red_delete":bool
  in  "font_red":bool
  in  "font_go":bool
  in  "font_delete":bool
  in  "font_colors":bool
  in  "font_add":bool
  in  "font":bool
  in  "folding_fan":bool
  in  "folders_explorer":bool
  in  "folders":bool
  in  "folder_wrench":bool
  in  "folder_vertical_zipper":bool
  in  "folder_vertical_torn":bool
  in  "folder_vertical_rename":bool
  in  "folder_vertical_open":bool
  in  "folder_vertical_document":bool
  in  "folder_user":bool
  in  "folder_torn":bool
  in  "folder_table":bool
  in  "folder_star":bool
  in  "folder_stand":bool
  in  "folder_search":bool
  in  "folder_red":bool
  in  "folder_picture":bool
  in  "folder_palette":bool
  in  "folder_page_white":bool
  in  "folder_page":bool
  in  "folder_link":bool
  in  "folder_lightbulb":bool
  in  "folder_key":bool
  in  "folder_image":bool
  in  "folder_heart":bool
  in  "folder_green":bool
  in  "folder_go":bool
  in  "folder_find":bool
  in  "folder_feed":bool
  in  "folder_explore":bool
  in  "folder_error":bool
  in  "folder_edit":bool
  in  "folder_delete":bool
  in  "folder_database":bool
  in  "folder_camera":bool
  in  "folder_bug":bool
  in  "folder_brick":bool
  in  "folder_blue":bool
  in  "folder_black":bool